vi "FlexMag - 23-03-2023.vi"() -> ()   [LabVIEW 2018] (continued)
        n5932 = Build Array(49152 ("element")) -> (w10400:i32[])
        n5933 = call "MB Serial Master Query Write Multiple Registers (poly).vi"("VISA resource name"=w10402, "Starting Address"=u16 320, "Registers"=w10400, "error in"=w10401, "Serial Parameters"=w10395) -> ("VISA resource name out"=w10406:refnum<visa-resource-name>, "error out"=w10407:errorcluster)  [unwired: 12 in, 1 out]
        n5934 = Build Array(49407 ("element")) -> (w10403:i32[])
        n5935 = call "MB Serial Master Query Write Multiple Registers (poly).vi"("VISA resource name"=w10406, "Starting Address"=u16 320, "Registers"=w10403, "error in"=w10407, "Serial Parameters"=w10395) -> ("VISA resource name out"=w10397:refnum<visa-resource-name>, "error out"=w10396:errorcluster)  [unwired: 12 in, 1 out]
      }
      frame 11 {
        w10417 = T15 {"Mode"=enum."RTU", "Slave Address"=1} ("Serial Parameters")
        n5936 = Type Cast(type=i16 0, x="TC2_AO1_bottom_limit_value") -> (*(type *) &x=w10409:i16)
        n5937 = Build Array(w10409) -> (w10410:i16[])
        n5938 = Increment(x=u16 166) -> (x+1=w10414:u16)
        n5939 = local write "TC2_AO1_bottom_limit_set"(FALSE ("TC2_AO1_bottom_limit_set")) -> ()
        n5940 = call "MB Serial Master Query Write Multiple Registers (poly).vi"("VISA resource name"=w10416, "Starting Address"=w10414, "Registers"=w10410, "error in"=w10415, "Serial Parameters"=w10417) -> ("VISA resource name out"=w10424:refnum<visa-resource-name>, "error out"=w10423:errorcluster)  [unwired: 12 in, 1 out]
        n5941 = Build Array(49152 ("element")) -> (w10422:i32[])
        n5942 = call "MB Serial Master Query Write Multiple Registers (poly).vi"("VISA resource name"=w10424, "Starting Address"=u16 320, "Registers"=w10422, "error in"=w10423, "Serial Parameters"=w10417) -> ("VISA resource name out"=w10428:refnum<visa-resource-name>, "error out"=w10429:errorcluster)  [unwired: 12 in, 1 out]
        n5943 = Build Array(49407 ("element")) -> (w10425:i32[])
        n5944 = call "MB Serial Master Query Write Multiple Registers (poly).vi"("VISA resource name"=w10428, "Starting Address"=u16 320, "Registers"=w10425, "error in"=w10429, "Serial Parameters"=w10417) -> ("VISA resource name out"=w10419:refnum<visa-resource-name>, "error out"=w10418:errorcluster)  [unwired: 12 in, 1 out]
      }
      frame 12 {
        w10439 = T15 {"Mode"=enum."RTU", "Slave Address"=1} ("Serial Parameters")
        n5945 = Type Cast(type=i16 0, x=sgl 0.0 ("TC1_AO1_bottom_limit_value 2")) -> (*(type *) &x=w10431:i16)
        n5946 = Build Array(w10431) -> (w10432:i16[])
        n5947 = Increment(x=u16 198) -> (x+1=w10436:u16)
        n5948 = local write "TC2_AO1_polarity(neg_to_pos)"(FALSE ("TC2_AO1_polarity(neg_to_pos)")) -> ()
        n5949 = call "MB Serial Master Query Write Multiple Registers (poly).vi"("VISA resource name"=w10438, "Starting Address"=w10436, "Registers"=w10432, "error in"=w10437, "Serial Parameters"=w10439) -> ("VISA resource name out"=w10446:refnum<visa-resource-name>, "error out"=w10445:errorcluster)  [unwired: 12 in, 1 out]
        n5950 = Build Array(49152 ("element")) -> (w10444:i32[])
        n5951 = call "MB Serial Master Query Write Multiple Registers (poly).vi"("VISA resource name"=w10446, "Starting Address"=u16 320, "Registers"=w10444, "error in"=w10445, "Serial Parameters"=w10439) -> ("VISA resource name out"=w10450:refnum<visa-resource-name>, "error out"=w10451:errorcluster)  [unwired: 12 in, 1 out]
        n5952 = Build Array(49407 ("element")) -> (w10447:i32[])
        n5953 = call "MB Serial Master Query Write Multiple Registers (poly).vi"("VISA resource name"=w10450, "Starting Address"=u16 320, "Registers"=w10447, "error in"=w10451, "Serial Parameters"=w10439) -> ("VISA resource name out"=w10441:refnum<visa-resource-name>, "error out"=w10440:errorcluster)  [unwired: 12 in, 1 out]
      }
      frame 13 {
        w10461 = T15 {"Mode"=enum."RTU", "Slave Address"=1} ("Serial Parameters")
        n5954 = Type Cast(type=i16 0, x=sgl 1.0 ("TC1_AO1_bottom_limit_value 2")) -> (*(type *) &x=w10453:i16)
        n5955 = Build Array(w10453) -> (w10454:i16[])
        n5956 = Increment(x=u16 198) -> (x+1=w10458:u16)
        n5957 = local write "TC2_AO1_polarity(pos_to_neg)"(FALSE ("TC2_AO1_polarity(pos_to_neg)")) -> ()
        n5958 = call "MB Serial Master Query Write Multiple Registers (poly).vi"("VISA resource name"=w10460, "Starting Address"=w10458, "Registers"=w10454, "error in"=w10459, "Serial Parameters"=w10461) -> ("VISA resource name out"=w10468:refnum<visa-resource-name>, "error out"=w10467:errorcluster)  [unwired: 12 in, 1 out]
        n5959 = Build Array(49152 ("element")) -> (w10466:i32[])
        n5960 = call "MB Serial Master Query Write Multiple Registers (poly).vi"("VISA resource name"=w10468, "Starting Address"=u16 320, "Registers"=w10466, "error in"=w10467, "Serial Parameters"=w10461) -> ("VISA resource name out"=w10472:refnum<visa-resource-name>, "error out"=w10473:errorcluster)  [unwired: 12 in, 1 out]
        n5961 = Build Array(49407 ("element")) -> (w10469:i32[])
        n5962 = call "MB Serial Master Query Write Multiple Registers (poly).vi"("VISA resource name"=w10472, "Starting Address"=u16 320, "Registers"=w10469, "error in"=w10473, "Serial Parameters"=w10461) -> ("VISA resource name out"=w10463:refnum<visa-resource-name>, "error out"=w10462:errorcluster)  [unwired: 12 in, 1 out]
      }
      frame 14 {
        w10483 = T15 {"Mode"=enum."RTU", "Slave Address"=1} ("Serial Parameters")
        n5963 = Type Cast(type=i16 0, x=sgl 2.0 ("TC1_AO1_bottom_limit_value 2")) -> (*(type *) &x=w10475:i16)
        n5964 = local write "TC2_display_tension_set"(FALSE ("TC2_display_tension")) -> ()
        n5965 = Build Array(w10475) -> (w10476:i16[])
        n5966 = Increment(x=u16 8) -> (x+1=w10480:u16)
        n5967 = call "MB Serial Master Query Write Multiple Registers (poly).vi"("VISA resource name"=w10482, "Starting Address"=w10480, "Registers"=w10476, "error in"=w10481, "Serial Parameters"=w10483) -> ("VISA resource name out"=w10490:refnum<visa-resource-name>, "error out"=w10489:errorcluster)  [unwired: 12 in, 1 out]
        n5968 = Build Array(49152 ("element")) -> (w10488:i32[])
        n5969 = call "MB Serial Master Query Write Multiple Registers (poly).vi"("VISA resource name"=w10490, "Starting Address"=u16 320, "Registers"=w10488, "error in"=w10489, "Serial Parameters"=w10483) -> ("VISA resource name out"=w10494:refnum<visa-resource-name>, "error out"=w10495:errorcluster)  [unwired: 12 in, 1 out]
        n5970 = Build Array(49407 ("element")) -> (w10491:i32[])
        n5971 = call "MB Serial Master Query Write Multiple Registers (poly).vi"("VISA resource name"=w10494, "Starting Address"=u16 320, "Registers"=w10491, "error in"=w10495, "Serial Parameters"=w10483) -> ("VISA resource name out"=w10485:refnum<visa-resource-name>, "error out"=w10484:errorcluster)  [unwired: 12 in, 1 out]
      }
      frame 15 {
        w10505 = T15 {"Mode"=enum."RTU", "Slave Address"=1} ("Serial Parameters")
        n5972 = Type Cast(type=i16 0, x=sgl 5.0 ("TC1_AO1_bottom_limit_value 2")) -> (*(type *) &x=w10497:i16)
        n5973 = Build Array(w10497) -> (w10498:i16[])
        n5974 = Increment(x=u16 8) -> (x+1=w10502:u16)
        n5975 = call "MB Serial Master Query Write Multiple Registers (poly).vi"("VISA resource name"=w10504, "Starting Address"=w10502, "Registers"=w10498, "error in"=w10503, "Serial Parameters"=w10505) -> ("VISA resource name out"=w10512:refnum<visa-resource-name>, "error out"=w10511:errorcluster)  [unwired: 12 in, 1 out]
        n5976 = local write "TC2_display_AO1_set"(FALSE ("TC2_display_tension")) -> ()
        n5977 = Build Array(49152 ("element")) -> (w10510:i32[])
        n5978 = call "MB Serial Master Query Write Multiple Registers (poly).vi"("VISA resource name"=w10512, "Starting Address"=u16 320, "Registers"=w10510, "error in"=w10511, "Serial Parameters"=w10505) -> ("VISA resource name out"=w10516:refnum<visa-resource-name>, "error out"=w10517:errorcluster)  [unwired: 12 in, 1 out]
        n5979 = Build Array(49407 ("element")) -> (w10513:i32[])
        n5980 = call "MB Serial Master Query Write Multiple Registers (poly).vi"("VISA resource name"=w10516, "Starting Address"=u16 320, "Registers"=w10513, "error in"=w10517, "Serial Parameters"=w10505) -> ("VISA resource name out"=w10507:refnum<visa-resource-name>, "error out"=w10506:errorcluster)  [unwired: 12 in, 1 out]
      }
      frame 16 {
        w10527 = T15 {"Mode"=enum."RTU", "Slave Address"=1} ("Serial Parameters")
        n5981 = Type Cast(type=i16 0, x=sgl 4.0 ("TC1_AO1_bottom_limit_value 2")) -> (*(type *) &x=w10519:i16)
        n5982 = local write "TC2_display_tension_actual"(FALSE ("TC2_display_tension")) -> ()
        n5983 = Build Array(w10519) -> (w10520:i16[])
        n5984 = Increment(x=u16 10) -> (x+1=w10524:u16)
        n5985 = call "MB Serial Master Query Write Multiple Registers (poly).vi"("VISA resource name"=w10526, "Starting Address"=w10524, "Registers"=w10520, "error in"=w10525, "Serial Parameters"=w10527) -> ("VISA resource name out"=w10534:refnum<visa-resource-name>, "error out"=w10533:errorcluster)  [unwired: 12 in, 1 out]
        n5986 = Build Array(49152 ("element")) -> (w10532:i32[])
        n5987 = call "MB Serial Master Query Write Multiple Registers (poly).vi"("VISA resource name"=w10534, "Starting Address"=u16 320, "Registers"=w10532, "error in"=w10533, "Serial Parameters"=w10527) -> ("VISA resource name out"=w10538:refnum<visa-resource-name>, "error out"=w10539:errorcluster)  [unwired: 12 in, 1 out]
        n5988 = Build Array(49407 ("element")) -> (w10535:i32[])
        n5989 = call "MB Serial Master Query Write Multiple Registers (poly).vi"("VISA resource name"=w10538, "Starting Address"=u16 320, "Registers"=w10535, "error in"=w10539, "Serial Parameters"=w10527) -> ("VISA resource name out"=w10529:refnum<visa-resource-name>, "error out"=w10528:errorcluster)  [unwired: 12 in, 1 out]
      }
      frame 17 {
        w10549 = T15 {"Mode"=enum."RTU", "Slave Address"=1} ("Serial Parameters")
        n5990 = Type Cast(type=i16 0, x=sgl 0.0 ("TC1_AO1_bottom_limit_value 2")) -> (*(type *) &x=w10541:i16)
        n5991 = Build Array(w10541) -> (w10542:i16[])
        n5992 = Increment(x=u16 10) -> (x+1=w10546:u16)
        n5993 = call "MB Serial Master Query Write Multiple Registers (poly).vi"("VISA resource name"=w10548, "Starting Address"=w10546, "Registers"=w10542, "error in"=w10547, "Serial Parameters"=w10549) -> ("VISA resource name out"=w10556:refnum<visa-resource-name>, "error out"=w10555:errorcluster)  [unwired: 12 in, 1 out]
        n5994 = local write "TC2_display_AO1_actual"(FALSE ("TC2_display_tension")) -> ()
        n5995 = Build Array(49152 ("element")) -> (w10554:i32[])
        n5996 = call "MB Serial Master Query Write Multiple Registers (poly).vi"("VISA resource name"=w10556, "Starting Address"=u16 320, "Registers"=w10554, "error in"=w10555, "Serial Parameters"=w10549) -> ("VISA resource name out"=w10560:refnum<visa-resource-name>, "error out"=w10561:errorcluster)  [unwired: 12 in, 1 out]
        n5997 = Build Array(49407 ("element")) -> (w10557:i32[])
        n5998 = call "MB Serial Master Query Write Multiple Registers (poly).vi"("VISA resource name"=w10560, "Starting Address"=u16 320, "Registers"=w10557, "error in"=w10561, "Serial Parameters"=w10549) -> ("VISA resource name out"=w10551:refnum<visa-resource-name>, "error out"=w10550:errorcluster)  [unwired: 12 in, 1 out]
      }
      frame 18 {
        n5999 = Build Array(i16 21767) -> (w10568:i16[])
        n6000 = call "MB Serial Master Query Write Multiple Registers (poly).vi"("VISA resource name"=w10570, "Starting Address"=u16 322 ("x"), "Registers"=w10568, "error in"=w10569, "Serial Parameters"=T15 {"Mode"=enum."RTU", "Slave Address"=1}) -> ("VISA resource name out"=w10563:refnum<visa-resource-name>, "error out"=w10564:errorcluster)  [unwired: 12 in, 1 out]
        n6001 = local write "TC2_tare_function"(FALSE ("TC2_tare_function")) -> ()
        n6002 = Build Array(49407 ("element")) -> (w10573:i32[])
        n6003 = call "MB Serial Master Query Write Multiple Registers (poly).vi"("VISA resource name"=w10563, "Starting Address"=u16 320, "Registers"=w10573, "error in"=w10564) -> ("VISA resource name out"=w10572:refnum<visa-resource-name>, "error out"=w10571:errorcluster)  [unwired: 13 in, 1 out]
      }
      frame 19 {
        w10594 = T15 {"Mode"=enum."RTU", "Slave Address"=1} ("Serial Parameters")
        n6004 = Build Array("TC2_regulation_type_value") -> (w10583:sgl[])
        n6005 = call "MB Serial Master Query Write Multiple Registers (poly).vi"("VISA resource name"=w10580, "Starting Address"=u16 107, "Registers"=w10583, "error in"=w10579, "Serial Parameters"=w10594) -> ("VISA resource name out"=w10592:refnum<visa-resource-name>, "error out"=w10593:errorcluster)  [unwired: 12 in, 1 out]
        n6006 = Build Array(49152 ("element")) -> (w10587:i32[])
        n6007 = local write "TC2_regulation_type_selection"(FALSE ("TC2_regulation_type_selection")) -> ()
        n6008 = call "MB Serial Master Query Write Multiple Registers (poly).vi"("VISA resource name"=w10592, "Starting Address"=u16 320, "Registers"=w10587, "error in"=w10593, "Serial Parameters"=w10594) -> ("VISA resource name out"=w10585:refnum<visa-resource-name>, "error out"=w10584:errorcluster)  [unwired: 12 in, 1 out]
        n6009 = Build Array(49407 ("element")) -> (w10586:i32[])
        n6010 = call "MB Serial Master Query Write Multiple Registers (poly).vi"("VISA resource name"=w10585, "Starting Address"=u16 320, "Registers"=w10586, "error in"=w10584, "Serial Parameters"=w10594) -> ("VISA resource name out"=w10581:refnum<visa-resource-name>, "error out"=w10578:errorcluster)  [unwired: 12 in, 1 out]
      }
      frame 20 {
        w10613 = T15 {"Mode"=enum."RTU", "Slave Address"=1} ("Serial Parameters")
        n6011 = Build Array("TC2_setpoint_type_value") -> (w10602:sgl[])
        n6012 = call "MB Serial Master Query Write Multiple Registers (poly).vi"("VISA resource name"=w10599, "Starting Address"=u16 141, "Registers"=w10602, "error in"=w10598, "Serial Parameters"=w10613) -> ("VISA resource name out"=w10611:refnum<visa-resource-name>, "error out"=w10612:errorcluster)  [unwired: 12 in, 1 out]
        n6013 = Build Array(49152 ("element")) -> (w10606:i32[])
        n6014 = call "MB Serial Master Query Write Multiple Registers (poly).vi"("VISA resource name"=w10611, "Starting Address"=u16 320, "Registers"=w10606, "error in"=w10612, "Serial Parameters"=w10613) -> ("VISA resource name out"=w10604:refnum<visa-resource-name>, "error out"=w10603:errorcluster)  [unwired: 12 in, 1 out]
        n6015 = local write "TC2_setpoint_type"(FALSE ("TC2_regulation_type_selection")) -> ()
        n6016 = Build Array(49407 ("element")) -> (w10605:i32[])
        n6017 = call "MB Serial Master Query Write Multiple Registers (poly).vi"("VISA resource name"=w10604, "Starting Address"=u16 320, "Registers"=w10605, "error in"=w10603, "Serial Parameters"=w10613) -> ("VISA resource name out"=w10600:refnum<visa-resource-name>, "error out"=w10597:errorcluster)  [unwired: 12 in, 1 out]
      }
      frame 21 {
        w10632 = T15 {"Mode"=enum."RTU", "Slave Address"=1} ("Serial Parameters")
        n6018 = Build Array("tc2 data set to reg") -> (w10621:sgl[])
        n6019 = call "MB Serial Master Query Write Multiple Registers (poly).vi"("VISA resource name"=w10619, "Starting Address"="tc2 Starting Address", "Registers"=w10621, "error in"=w10618, "Serial Parameters"=w10632) -> ("VISA resource name out"=w10630:refnum<visa-resource-name>, "error out"=w10631:errorcluster)  [unwired: 12 in, 1 out]
        n6020 = Build Array(49152 ("element")) -> (w10625:i32[])
        n6021 = call "MB Serial Master Query Write Multiple Registers (poly).vi"("VISA resource name"=w10630, "Starting Address"=u16 320, "Registers"=w10625, "error in"=w10631, "Serial Parameters"=w10632) -> ("VISA resource name out"=w10623:refnum<visa-resource-name>, "error out"=w10622:errorcluster)  [unwired: 12 in, 1 out]
        n6022 = local write "TC2_reg_set"(FALSE ("TC2_regulation_type_selection")) -> ()
        n6023 = Build Array(49407 ("element")) -> (w10624:i32[])
        n6024 = call "MB Serial Master Query Write Multiple Registers (poly).vi"("VISA resource name"=w10623, "Starting Address"=u16 320, "Registers"=w10624, "error in"=w10622, "Serial Parameters"=w10632) -> ("VISA resource name out"=w10620:refnum<visa-resource-name>, "error out"=w10617:errorcluster)  [unwired: 12 in, 1 out]
      }
    }
  }
  n6025 = while {
    tunnel: w45 -> [w11141]
    tunnel: w44 -> [w11140]
    tunnel: [w11139] -> w43
    tunnel: [w11138] -> w42
    stop <- FALSE stop-if-true
    n6026 = Wait Until Next ms Multiple(millisecond multiple=u32 300) -> ()  [unwired: 1 out]
    n6027 = case shown="False" "Counter data set" {
      tunnel: w11141 -> [w11149 w11158]
      tunnel: [w11148 w11157] -> w11139
      tunnel: [w11147 w11156] -> w11138
      tunnel: w11140 -> [w11143 _]
      frame False {
        n6028 = call-poly "MB Serial Master Query (poly).vi"("VISA resource name"=w11149, "Starting Address"=u16 1000, "Quantity"=u16 13, "error in"=w11143, "Serial Parameters"=T15 {"Mode"=enum."RTU", "Slave Address"=1}) -> ("VISA resource name out"=w11148:refnum<visa-resource-name>, "Input Registers"=w11146:u16[], "error out"=w11147:errorcluster)  [unwired: 1 in, 11 out]
        n6029 = Index Array(array=w11146, index=3) -> (element=→"Counter Read Data":u16)
      }
      frame True {
        n6030 = local write "Counter data set"(FALSE ("Counter_reset")) -> ()
        n6031 = call-poly "MB Serial Master Query (poly).vi"("VISA resource name"=w11158, "Address"="Counter Data set", "Coil"=TRUE, "Serial Parameters"=T15 {"Mode"=enum."RTU", "Slave Address"=1}) -> ("VISA resource name out"=w11157:refnum<visa-resource-name>, "error out"=w11156:errorcluster)  [unwired: 2 in, 12 out]
      }
    }
  }
  n6032 = while {
    tunnel: w27 -> [w11175]
    tunnel: w26 -> [w11174]
    tunnel: [w11172] -> w28
    tunnel: [w11171] -> w29
    stop <- FALSE stop-if-true
    n6033 = Compound Arithmetic op=OR("MWPS1 open", "MWPS1 auto open") -> (w11161:bool)
    n6034 = Compound Arithmetic op=OR("MWPS1 close", "MWPS1 auto close") -> (w11160:bool)
    n6035 = Wait Until Next ms Multiple(millisecond multiple=u32 300) -> ()  [unwired: 1 out]
    n6036 = Build Array(FALSE, w11161, w11160) -> (w11168:bool[])
    n6037 = Boolean Array To Number(Boolean array=w11168) -> (number=w11167:u32)
    n6038 = Mantissa & Exponent(0:w11167) -> (2:w11166:dbl)  [unwired: 1 out]
    n6039 = case shown="1" w11166 {
      tunnel: w11175 -> [w11190 w11222 w11242]
      tunnel: w11174 -> [w11189 w11221 w11241]
      tunnel: [w11188 w11212 w11232] -> w11172
      tunnel: [w11187 w11211 w11231] -> w11171
      frame 0, Default {
        n6040 = VISA Write(VISA resource name=w11190, write buffer="\u0000%\u0000%", error in (no error)=w11189) -> (VISA resource name out=w11186:refnum<visa-resource-name>, error out=w11185:errorcluster)  [unwired: 1 out]
        n6041 = property class="Instr"(reference=w11186, error in=w11185) -> (reference out=w11184:refnum<visa-resource-name>, error out=w11183:errorcluster, "Serial Settings:Number of Bytes at Serial Port"=w11182:u32)
        n6042 = stacked-sequence {
          tunnel: [w11194] -> w11181
          tunnel: w11184 -> [w11194]
          tunnel: [w11193] -> w11180
          tunnel: w11183 -> [w11193]
          tunnel: [w11192] -> w11179
          tunnel: w11182 -> [w11192]
          tunnel: "microwave1 wait ms" -> [w11191]
          frame #0 {
            n6043 = Wait (ms)(milliseconds to wait=w11191) -> ()  [unwired: 1 out]
          }
        }
        n6044 = VISA Read(VISA resource name=w11181, byte count=w11179, error in (no error)=w11180) -> (VISA resource name out=w11188:refnum<visa-resource-name>, read buffer=→"microwave1 read":string, error out=w11187:errorcluster)  [unwired: 1 out]
      }
      frame 1 {
        n6045 = stacked-sequence {
          frame #0 {
            n6046 = Wait (ms)(milliseconds to wait=u32 200) -> ()  [unwired: 1 out]
          }
          frame #1 {
            n6047 = local write "MWPS1 auto open"(FALSE ("Mwps_auto_open")) -> ()
          }
        }
        n6048 = Divide(x="MWPS1 set", y=10.0) -> (x/y=w11205:dbl)
        n6049 = Add(x=w11205, y=165.0 ("Mwps_set 2")) -> (x+y=w11199:dbl)
        n6050 = Greater?(x=w11199, y=256.0) -> (0:w11203:bool)
        n6051 = Subtract(x=w11199, y=256.0) -> (x-y=w11200:dbl)
        n6052 = Select(t=w11200, s=w11203, f=w11199) -> (s? t:f=w11197:dbl)
        n6053 = Build Array(w11205) -> (w11209:dbl[])
        n6054 = Build Array(w11197) -> (w11198:dbl[])
        n6055 = Byte Array To String(unsigned byte array=w11209) -> (string=w11208:string)
        n6056 = Byte Array To String(unsigned byte array=w11198) -> (string=w11196:string)
        n6057 = Concatenate Strings("€%" ("write buffer"), w11208, w11196) -> (w11195:string)
        n6058 = VISA Write(VISA resource name=w11222, write buffer=w11195, error in (no error)=w11221) -> (VISA resource name out=w11220:refnum<visa-resource-name>, error out=w11219:errorcluster)  [unwired: 1 out]
        n6059 = property class="Instr"(reference=w11220, error in=w11219) -> (reference out=w11218:refnum<visa-resource-name>, error out=w11217:errorcluster, "Serial Settings:Number of Bytes at Serial Port"=w11216:u32)
        n6060 = stacked-sequence {
          tunnel: [w11228] -> w11215
          tunnel: w11218 -> [w11228]
          tunnel: [w11227] -> w11214
          tunnel: w11217 -> [w11227]
          tunnel: [w11226] -> w11213
          tunnel: w11216 -> [w11226]
          frame #0 {
            n6061 = Wait (ms)(milliseconds to wait=u32 300) -> ()  [unwired: 1 out]
          }
        }
        n6062 = VISA Read(VISA resource name=w11215, byte count=w11213, error in (no error)=w11214) -> (VISA resource name out=w11212:refnum<visa-resource-name>, error out=w11211:errorcluster)  [unwired: 2 out]
      }
      frame 2 {
        n6063 = stacked-sequence {
          frame #0 {
            n6064 = Wait (ms)(milliseconds to wait=u32 200) -> ()  [unwired: 1 out]
          }
          frame #1 {
            n6065 = local write "MWPS1 auto close"(FALSE ("Mwps_auto_open")) -> ()
          }
        }
        n6066 = local write "MWPS1 set"(0.0 ("Mwps_set")) -> ()
        n6067 = VISA Write(VISA resource name=w11242, write buffer="€%\u0000¥", error in (no error)=w11241) -> (VISA resource name out=w11240:refnum<visa-resource-name>, error out=w11239:errorcluster)  [unwired: 1 out]
        n6068 = property class="Instr"(reference=w11240, error in=w11239) -> (reference out=w11238:refnum<visa-resource-name>, error out=w11237:errorcluster, "Serial Settings:Number of Bytes at Serial Port"=w11236:u32)
        n6069 = stacked-sequence {
          tunnel: [w11248] -> w11235
          tunnel: w11238 -> [w11248]
          tunnel: [w11247] -> w11234
          tunnel: w11237 -> [w11247]
          tunnel: [w11246] -> w11233
          tunnel: w11236 -> [w11246]
          frame #0 {
            n6070 = Wait (ms)(milliseconds to wait=u32 300) -> ()  [unwired: 1 out]
          }
        }
        n6071 = VISA Read(VISA resource name=w11235, byte count=w11233, error in (no error)=w11234) -> (VISA resource name out=w11232:refnum<visa-resource-name>, error out=w11231:errorcluster)  [unwired: 2 out]
      }
    }
  }
  n6072 = while {
    tunnel: w24 -> [w11264]
    tunnel: w25 -> [w11263]
    tunnel: [w11261] -> w22
    tunnel: [w11260] -> w23
    stop <- FALSE stop-if-true
    n6073 = Wait Until Next ms Multiple(millisecond multiple=u32 300) -> ()  [unwired: 1 out]
    n6074 = Compound Arithmetic op=OR("MWPS2 open", "MWPS2 auto open") -> (w11249:bool)
    n6075 = Compound Arithmetic op=OR("MWPS2 close", "MWPS2 auto close") -> (w11250:bool)
    n6076 = Build Array(FALSE, w11249, w11250) -> (w11257:bool[])
    n6077 = Boolean Array To Number(Boolean array=w11257) -> (number=w11256:u32)
    n6078 = Mantissa & Exponent(0:w11256) -> (2:w11255:dbl)  [unwired: 1 out]
    n6079 = case shown="0, Default" w11255 {
      tunnel: w11264 -> [w11279 w11311 w11331]
      tunnel: w11263 -> [w11278 w11310 w11330]
      tunnel: [w11277 w11301 w11321] -> w11261
      tunnel: [w11276 w11300 w11320] -> w11260
      frame 0, Default {
        n6080 = VISA Write(VISA resource name=w11279, write buffer="\u0000%\u0000%", error in (no error)=w11278) -> (VISA resource name out=w11275:refnum<visa-resource-name>, error out=w11274:errorcluster)  [unwired: 1 out]
        n6081 = property class="Instr"(reference=w11275, error in=w11274) -> (reference out=w11273:refnum<visa-resource-name>, error out=w11272:errorcluster, "Serial Settings:Number of Bytes at Serial Port"=w11271:u32)
        n6082 = stacked-sequence {
          tunnel: [w11283] -> w11270
          tunnel: w11273 -> [w11283]
          tunnel: [w11282] -> w11269
          tunnel: w11272 -> [w11282]
          tunnel: [w11281] -> w11268
          tunnel: w11271 -> [w11281]
          tunnel: "microwave2 wait ms" -> [w11280]
          frame #0 {
            n6083 = Wait (ms)(milliseconds to wait=w11280) -> ()  [unwired: 1 out]
          }
        }
        n6084 = VISA Read(VISA resource name=w11270, byte count=w11268, error in (no error)=w11269) -> (VISA resource name out=w11277:refnum<visa-resource-name>, read buffer=→"microwave2 read":string, error out=w11276:errorcluster)  [unwired: 1 out]
      }
      frame 1 {
        n6085 = stacked-sequence {
          frame #0 {
            n6086 = Wait (ms)(milliseconds to wait=u32 200) -> ()  [unwired: 1 out]
          }
          frame #1 {
            n6087 = local write "MWPS2 auto open"(FALSE ("Mwps_auto_open")) -> ()
          }
        }
        n6088 = Divide(x="MWPS2 set", y=10.0) -> (x/y=w11294:dbl)
        n6089 = Add(x=w11294, y=165.0 ("Mwps_set 2")) -> (x+y=w11288:dbl)
        n6090 = Greater?(x=w11288, y=256.0) -> (0:w11292:bool)
        n6091 = Subtract(x=w11288, y=256.0) -> (x-y=w11289:dbl)
        n6092 = Select(t=w11289, s=w11292, f=w11288) -> (s? t:f=w11286:dbl)
        n6093 = Build Array(w11294) -> (w11298:dbl[])
        n6094 = Build Array(w11286) -> (w11287:dbl[])
        n6095 = Byte Array To String(unsigned byte array=w11298) -> (string=w11297:string)
        n6096 = Byte Array To String(unsigned byte array=w11287) -> (string=w11285:string)
        n6097 = Concatenate Strings("€%" ("write buffer"), w11297, w11285) -> (w11284:string)
        n6098 = VISA Write(VISA resource name=w11311, write buffer=w11284, error in (no error)=w11310) -> (VISA resource name out=w11309:refnum<visa-resource-name>, error out=w11308:errorcluster)  [unwired: 1 out]
        n6099 = property class="Instr"(reference=w11309, error in=w11308) -> (reference out=w11307:refnum<visa-resource-name>, error out=w11306:errorcluster, "Serial Settings:Number of Bytes at Serial Port"=w11305:u32)
        n6100 = stacked-sequence {
          tunnel: [w11317] -> w11304
          tunnel: w11307 -> [w11317]
          tunnel: [w11316] -> w11303
          tunnel: w11306 -> [w11316]
          tunnel: [w11315] -> w11302
          tunnel: w11305 -> [w11315]
          frame #0 {
            n6101 = Wait (ms)(milliseconds to wait=u32 300) -> ()  [unwired: 1 out]
          }
        }
        n6102 = VISA Read(VISA resource name=w11304, byte count=w11302, error in (no error)=w11303) -> (VISA resource name out=w11301:refnum<visa-resource-name>, error out=w11300:errorcluster)  [unwired: 2 out]
      }
      frame 2 {
        n6103 = stacked-sequence {
          frame #0 {
            n6104 = Wait (ms)(milliseconds to wait=u32 200) -> ()  [unwired: 1 out]
          }
          frame #1 {
            n6105 = local write "MWPS2 auto close"(FALSE ("Mwps_auto_open")) -> ()
          }
        }
        n6106 = local write "MWPS2 set"(0.0 ("Mwps_set")) -> ()
        n6107 = VISA Write(VISA resource name=w11331, write buffer="€%\u0000¥", error in (no error)=w11330) -> (VISA resource name out=w11329:refnum<visa-resource-name>, error out=w11328:errorcluster)  [unwired: 1 out]
        n6108 = property class="Instr"(reference=w11329, error in=w11328) -> (reference out=w11327:refnum<visa-resource-name>, error out=w11326:errorcluster, "Serial Settings:Number of Bytes at Serial Port"=w11325:u32)
        n6109 = stacked-sequence {
          tunnel: [w11337] -> w11324
          tunnel: w11327 -> [w11337]
          tunnel: [w11336] -> w11323
          tunnel: w11326 -> [w11336]
          tunnel: [w11335] -> w11322
          tunnel: w11325 -> [w11335]
          frame #0 {
            n6110 = Wait (ms)(milliseconds to wait=u32 300) -> ()  [unwired: 1 out]
          }
        }
        n6111 = VISA Read(VISA resource name=w11324, byte count=w11322, error in (no error)=w11323) -> (VISA resource name out=w11321:refnum<visa-resource-name>, error out=w11320:errorcluster)  [unwired: 2 out]
      }
    }
  }
  n6112 = while {
    tunnel: w58 -> [w11763]
    tunnel: w59 -> [w11762]
    shift-right: [w11588] -> _
    shift-left: _ -> [w11587]
    tunnel: [w11511] -> w60
    tunnel: [w11510] -> w61
    stop <- FALSE stop-if-true
    w11401 = "\b—"
    w11363 = "\b¢"
    # "guc kaynagı ACK gelınceye kadar bekler."
    # "ACK karsılıgı 06(hex) dır."
    n6113 = Tick Count (ms)() -> (millisecond timer value=w11588:u32)
    n6114 = Or(x="set rf", y="RF_auto_set") -> (x .or. y?=w11347:bool)
    n6115 = Or(x="RF on", y="RF_auto_on") -> (x .or. y?=w11358:bool)
    n6116 = Or(x="oto tuner", y="RF_auto_tuner") -> (x .or. y?=w11339:bool)
    n6117 = Or(x="RF off", y="RF_auto_off") -> (x .or. y?=w11356:bool)
    n6118 = Or(x="RF host", y="RF_auto_host") -> (x .or. y?=w11353:bool)
    n6119 = Subtract(x=w11588, y=w11587) -> (x-y=→"x-y":u32)
    n6120 = Or(x="Ramp Up time", y="Ramp Up time_auto") -> (x .or. y?=w11351:bool)
    n6121 = Boolean To (0,1)(Boolean=w11353) -> (0, 1=w11737:i16)
    n6122 = Boolean To (0,1)(Boolean=w11356) -> (0, 1=w11738:i16)
    n6123 = Boolean To (0,1)(Boolean=w11358) -> (0, 1=w11744:i16)
    n6124 = Boolean To (0,1)(Boolean=w11347) -> (0, 1=w11743:i16)
    n6125 = Boolean To (0,1)(Boolean=w11339) -> (0, 1=w11742:i16)
    n6126 = Boolean To (0,1)(Boolean="initialize") -> (0, 1=w11740:i16)
    n6127 = Boolean To (0,1)(Boolean="Load") -> (0, 1=w11465:i16)
    n6128 = Boolean To (0,1)(Boolean="Forward") -> (0, 1=w11462:i16)
    n6129 = Boolean To (0,1)(Boolean="External") -> (0, 1=w11468:i16)
    n6130 = Boolean To (0,1)(Boolean="Pulsing_off") -> (0, 1=w11475:i16)
    n6131 = Boolean To (0,1)(Boolean="internal") -> (0, 1=w11476:i16)
    n6132 = Boolean To (0,1)(Boolean="external") -> (0, 1=w11478:i16)
    n6133 = Boolean To (0,1)(Boolean="set duty") -> (0, 1=w11491:i16)
    n6134 = Boolean To (0,1)(Boolean=w11351) -> (0, 1=w11450:i16)
    n6135 = Boolean To (0,1)(Boolean="manuel tuner") -> (0, 1=w11741:i16)
    n6136 = Boolean To (0,1)(Boolean="set cap pos") -> (0, 1=w11739:i16)
    n6137 = Boolean To (0,1)(Boolean="set seri cap pos 2") -> (0, 1=w11736:i16)
    n6138 = Boolean To (0,1)(Boolean="set frequency") -> (0, 1=w11487:i16)
    n6139 = Multiply(x=w11737, y=i16 1) -> (x*y=w11460:i16)
    n6140 = Multiply(x=w11738, y=i16 3) -> (x*y=w11757:i16)
    n6141 = Multiply(x=w11744, y=i16 4) -> (x*y=w11758:i16)
    n6142 = Multiply(x=w11743, y=i16 5) -> (x*y=w11755:i16)
    n6143 = Multiply(x=w11742, y=i16 6) -> (x*y=w11753:i16)
    n6144 = Multiply(x=w11740, y=i16 8) -> (x*y=w11749:i16)
    n6145 = Or(x="Ramp down time", y="Ramp Down time_auto") -> (x .or. y?=w11346:bool)
    n6146 = Boolean To (0,1)(Boolean=w11346) -> (0, 1=w11448:i16)
    n6147 = Multiply(x=w11741, y=i16 7) -> (x*y=w11751:i16)
    n6148 = Multiply(x=w11739, y=i16 9) -> (x*y=w11747:i16)
    n6149 = Multiply(x=w11465, y=i16 2) -> (x*y=w11485:i16)
    n6150 = Multiply(x=w11736, y=i16 10) -> (x*y=w11745:i16)
    n6151 = Multiply(x=w11462, y=i16 11) -> (x*y=w11484:i16)
    n6152 = Multiply(x=w11468, y=i16 12) -> (x*y=w11483:i16)
    n6153 = Multiply(x=w11475, y=i16 13) -> (x*y=w11480:i16)
    n6154 = Multiply(x=w11476, y=i16 14) -> (x*y=w11481:i16)
    n6155 = Multiply(x=w11478, y=i16 15) -> (x*y=w11482:i16)
    n6156 = Multiply(x=w11487, y=i16 16) -> (x*y=w11489:i16)
    n6157 = Multiply(x=w11491, y=i16 17) -> (x*y=w11493:i16)
    n6158 = Multiply(x=w11450, y=i16 18) -> (x*y=w11447:i16)
    n6159 = Multiply(x=w11448, y=i16 19) -> (x*y=w11446:i16)
    n6160 = String To Byte Array(string=w11363) -> (unsigned byte array=w11445:u8[])
    n6161 = for {
      tunnel: w11445 -> [w11799] mode=indexing
      shift-right: [w11797] -> w11443
      shift-left: 0 -> [w11798]
      n6162 = Exclusive Or(1:w11798, 2:w11799) -> (0:w11797:i32)
    }
    n6163 = Wait Until Next ms Multiple(millisecond multiple=u32 300) -> ()  [unwired: 1 out]
    n6164 = Compound Arithmetic op=ADD(w11485, w11484, w11483, w11480, w11481, w11482, w11489, w11493) -> (w11461:i16)
    n6165 = Build Array(w11443) -> (w11442:i32[])
    n6166 = Compound Arithmetic op=ADD(w11460, w11757, w11758, w11755, w11753, w11751, w11749, w11747, w11745, w11461, w11447, w11446) -> (w11733:i16)
    n6167 = Byte Array To String(unsigned byte array=w11442) -> (string=w11441:string)
    n6168 = case shown="5" w11733 {
      tunnel: [w11910 w11914 w11919 w11933 w11939 w11946 w11969 w11986 w12002 w12022 w12047 w12063 w12077 w12091 w12105 w12119 w12133 w12161 w12180 w12206] -> w11735
      tunnel: [w11909 w11913 w11918 w11934 w11940 w11947 w11968 w11985 w12003 w12021 w12046 w12062 w12076 w12090 w12104 w12118 w12132 w12160 w12179 w12205] -> w11734
      tunnel: w11763 -> [w11910 w11912 w11921 w11936 w11942 w11949 w11971 w11988 w12001 w12024 w12049 w12065 w12079 w12093 w12107 w12121 w12135 w12163 w12182 w12208]
      tunnel: w11762 -> [w11909 w11911 w11920 w11935 w11941 w11948 w11970 w11987 w12000 w12023 w12048 w12064 w12078 w12092 w12106 w12120 w12134 w12162 w12181 w12207]
      frame 0, Default {
      }
      frame 1 {
        # "Host kontrol"
        n6169 = flat-sequence {
          frame #0 {
            n6170 = Wait (ms)(milliseconds to wait=u32 200) -> ()  [unwired: 1 out]
          }
          frame #1 {
            n6171 = local write "RF_auto_host"(FALSE ("RF_host_auto")) -> ()
          }
        }
        n6172 = VISA Write(VISA resource name=w11912, write buffer="\t\u000e\u0002\u0005", error in (no error)=w11911) -> (VISA resource name out=w11914:refnum<visa-resource-name>, error out=w11913:errorcluster)  [unwired: 1 out]
      }
      frame 2 {
        w11928 = "\t\u0003\u0007"
        n6173 = String To Byte Array(string=w11928) -> (unsigned byte array=w11922:u8[])
        n6174 = for {
          tunnel: w11922 -> [w11931] mode=indexing
          shift-right: [w11929] -> w11924
          shift-left: 0 -> [w11930]
          n6175 = Exclusive Or(1:w11930, 2:w11931) -> (0:w11929:i32)
        }
        n6176 = Build Array(w11924) -> (w11926:i32[])
        n6177 = Byte Array To String(unsigned byte array=w11926) -> (string=w11925:string)
        n6178 = Concatenate Strings(w11928, w11925) -> (w11927:string)
        n6179 = VISA Write(VISA resource name=w11921, write buffer=w11927, error in (no error)=w11920) -> (VISA resource name out=w11919:refnum<visa-resource-name>, error out=w11918:errorcluster)  [unwired: 1 out]
      }
      frame 3 {
        # "RF OFF"
        n6180 = local write "RF_auto_off"(FALSE ("RF_auto_off")) -> ()
        n6181 = VISA Write(VISA resource name=w11936, write buffer="\b\u0001\t", error in (no error)=w11935) -> (VISA resource name out=w11933:refnum<visa-resource-name>, error out=w11934:errorcluster)  [unwired: 1 out]
      }
      frame 4 {
        # "RF ON"
        n6182 = local write "RF_auto_on"(FALSE ("RF_auto_on")) -> ()
        n6183 = VISA Write(VISA resource name=w11942, write buffer="\b\u0002\n", error in (no error)=w11941) -> (VISA resource name out=w11939:refnum<visa-resource-name>, error out=w11940:errorcluster)  [unwired: 1 out]
      }
      frame 5 {
        n6184 = Quotient & Remainder(x="RF_forward_power_1", y=256.0) -> (x-y*floor(x/y)=w11956:dbl, floor(x/y)=w11952:dbl)
        n6185 = Build Array(w11956) -> (w11955:dbl[])
        n6186 = Build Array(w11952) -> (w11953:dbl[])
        n6187 = Byte Array To String(unsigned byte array=w11955) -> (string=w11954:string)
        n6188 = Byte Array To String(unsigned byte array=w11953) -> (string=w11951:string)
        n6189 = Concatenate Strings("\n\b", w11954, w11951) -> (w11958:string)
        n6190 = String To Byte Array(string=w11958) -> (unsigned byte array=w11964:u8[])
        n6191 = for {
          tunnel: w11964 -> [w11967] mode=indexing
          shift-right: [w11965] -> w11962
          shift-left: 0 -> [w11966]
          n6192 = Exclusive Or(1:w11966, 2:w11967) -> (0:w11965:i32)
        }
        n6193 = local write "RF_auto_set"(FALSE ("RF set auto")) -> ()
        n6194 = Build Array(w11962) -> (w11961:i32[])
        n6195 = Byte Array To String(unsigned byte array=w11961) -> (string=w11959:string)
        n6196 = Concatenate Strings(w11958, w11959) -> (w11950:string)
        n6197 = VISA Write(VISA resource name=w11949, write buffer=w11950, error in (no error)=w11948) -> (VISA resource name out=w11946:refnum<visa-resource-name>, error out=w11947:errorcluster)  [unwired: 1 out]
      }
      frame 6 {
        n6198 = Concatenate Strings("\t\r\u0001") -> (w11973:string)
        n6199 = String To Byte Array(string=w11973) -> (unsigned byte array=w11979:u8[])
        n6200 = flat-sequence {
          frame #0 {
            n6201 = Wait (ms)(milliseconds to wait=u32 200) -> ()  [unwired: 1 out]
          }
          frame #1 {
            n6202 = local write "RF_auto_tuner"(FALSE ("RF_auto_tuner")) -> ()
          }
        }
        n6203 = for {
          tunnel: w11979 -> [w11984] mode=indexing
          shift-right: [w11982] -> w11977
          shift-left: 0 -> [w11983]
          n6204 = Exclusive Or(1:w11983, 2:w11984) -> (0:w11982:i32)
        }
        n6205 = Build Array(w11977) -> (w11976:i32[])
        n6206 = Byte Array To String(unsigned byte array=w11976) -> (string=w11974:string)
        n6207 = Concatenate Strings(w11973, w11974) -> (w11972:string)
        n6208 = VISA Write(VISA resource name=w11971, write buffer=w11972, error in (no error)=w11970) -> (VISA resource name out=w11969:refnum<visa-resource-name>, error out=w11968:errorcluster)  [unwired: 1 out]
      }
      frame 7 {
        n6209 = Concatenate Strings("\t\r\u0000") -> (w11990:string)
        n6210 = String To Byte Array(string=w11990) -> (unsigned byte array=w11996:u8[])
        n6211 = for {
          tunnel: w11996 -> [w11999] mode=indexing
          shift-right: [w11997] -> w11994
          shift-left: 0 -> [w11998]
          n6212 = Exclusive Or(1:w11998, 2:w11999) -> (0:w11997:i32)
        }
        n6213 = Build Array(w11994) -> (w11993:i32[])
        n6214 = Byte Array To String(unsigned byte array=w11993) -> (string=w11991:string)
        n6215 = Concatenate Strings(w11990, w11991) -> (w11989:string)
        n6216 = VISA Write(VISA resource name=w11988, write buffer=w11989, error in (no error)=w11987) -> (VISA resource name out=w11986:refnum<visa-resource-name>, error out=w11985:errorcluster)  [unwired: 1 out]
      }
      frame 8 {
        w12007 = "\bo"
        n6217 = String To Byte Array(string=w12007) -> (unsigned byte array=w12010:u8[])
        n6218 = for {
          tunnel: w12010 -> [w12013] mode=indexing
          shift-right: [w12011] -> w12008
          shift-left: 0 -> [w12012]
          n6219 = Exclusive Or(1:w12012, 2:w12013) -> (0:w12011:i32)
        }
        n6220 = Build Array(w12008) -> (w12005:i32[])
        n6221 = Byte Array To String(unsigned byte array=w12005) -> (string=w12006:string)
        n6222 = Concatenate Strings(w12007, w12006) -> (w12004:string)
        n6223 = VISA Write(VISA resource name=w12001, write buffer=w12004, error in (no error)=w12000) -> (VISA resource name out=w12002:refnum<visa-resource-name>, error out=w12003:errorcluster)  [unwired: 1 out]
      }
      frame 9 {
        n6224 = Multiply(x="Set CL Position:", y=10.0) -> (x*y=w12016:dbl)
        n6225 = To Unsigned Long Integer(number=w12016) -> (unsigned 32bit integer=w12015:u32)
        n6226 = Quotient & Remainder(x=w12015, y=u32 256) -> (x-y*floor(x/y)=w12020:u32, floor(x/y)=w12019:u32)
        n6227 = Build Array(w12020, w12019) -> (w12027:u32[])
        n6228 = Byte Array To String(unsigned byte array=w12027) -> (string=w12026:string)
        n6229 = Concatenate Strings("\np", w12026) -> (w12028:string)
        n6230 = String To Byte Array(string=w12028) -> (unsigned byte array=w12034:u8[])
        n6231 = for {
          tunnel: w12034 -> [w12037] mode=indexing
          shift-right: [w12035] -> w12032
          shift-left: 0 -> [w12036]
          n6232 = Exclusive Or(1:w12036, 2:w12037) -> (0:w12035:i32)
        }
        n6233 = Build Array(w12032) -> (w12031:i32[])
        n6234 = Byte Array To String(unsigned byte array=w12031) -> (string=w12029:string)
        n6235 = Concatenate Strings(w12028, w12029) -> (w12025:string)
        n6236 = VISA Write(VISA resource name=w12024, write buffer=w12025, error in (no error)=w12023) -> (VISA resource name out=w12022:refnum<visa-resource-name>, error out=w12021:errorcluster)  [unwired: 1 out]
      }
      frame 10 {
        n6237 = Multiply(x="Set CT Position:", y=10.0) -> (x*y=w12038:dbl)
        n6238 = To Unsigned Long Integer(number=w12038) -> (unsigned 32bit integer=w12039:u32)
        n6239 = Quotient & Remainder(x=w12039, y=u32 256) -> (x-y*floor(x/y)=w12044:u32, floor(x/y)=w12043:u32)
        n6240 = Build Array(w12044, w12043) -> (w12041:u32[])
        n6241 = Byte Array To String(unsigned byte array=w12041) -> (string=w12051:string)
        n6242 = Concatenate Strings("\nz", w12051) -> (w12052:string)
        n6243 = String To Byte Array(string=w12052) -> (unsigned byte array=w12058:u8[])
        n6244 = for {
          tunnel: w12058 -> [w12061] mode=indexing
          shift-right: [w12059] -> w12056
          shift-left: 0 -> [w12060]
          n6245 = Exclusive Or(1:w12060, 2:w12061) -> (0:w12059:i32)
        }
        n6246 = Build Array(w12056) -> (w12055:i32[])
        n6247 = Byte Array To String(unsigned byte array=w12055) -> (string=w12053:string)
        n6248 = Concatenate Strings(w12052, w12053) -> (w12050:string)
        n6249 = VISA Write(VISA resource name=w12049, write buffer=w12050, error in (no error)=w12048) -> (VISA resource name out=w12047:refnum<visa-resource-name>, error out=w12046:errorcluster)  [unwired: 1 out]
      }
      frame 11 {
        w12069 = "\t\u0003\u0006"
        n6250 = String To Byte Array(string=w12069) -> (unsigned byte array=w12066:u8[])
        n6251 = for {
          tunnel: w12066 -> [w12075] mode=indexing
          shift-right: [w12073] -> w12068
          shift-left: 0 -> [w12074]
          n6252 = Exclusive Or(1:w12074, 2:w12075) -> (0:w12073:i32)
        }
        n6253 = Build Array(w12068) -> (w12070:i32[])
        n6254 = Byte Array To String(unsigned byte array=w12070) -> (string=w12071:string)
        n6255 = Concatenate Strings(w12069, w12071) -> (w12072:string)
        n6256 = VISA Write(VISA resource name=w12065, write buffer=w12072, error in (no error)=w12064) -> (VISA resource name out=w12063:refnum<visa-resource-name>, error out=w12062:errorcluster)  [unwired: 1 out]
      }
      frame 12 {
        w12084 = "\t\u0003\b"
        n6257 = String To Byte Array(string=w12084) -> (unsigned byte array=w12080:u8[])
        n6258 = for {
          tunnel: w12080 -> [w12089] mode=indexing
          shift-right: [w12087] -> w12082
          shift-left: 0 -> [w12088]
          n6259 = Exclusive Or(1:w12088, 2:w12089) -> (0:w12087:i32)
        }
        n6260 = Build Array(w12082) -> (w12083:i32[])
        n6261 = Byte Array To String(unsigned byte array=w12083) -> (string=w12085:string)
        n6262 = Concatenate Strings(w12084, w12085) -> (w12086:string)
        n6263 = VISA Write(VISA resource name=w12079, write buffer=w12086, error in (no error)=w12078) -> (VISA resource name out=w12077:refnum<visa-resource-name>, error out=w12076:errorcluster)  [unwired: 1 out]
      }
      frame 13 {
        w12098 = "\t\u001b\u0000"
        n6264 = String To Byte Array(string=w12098) -> (unsigned byte array=w12094:u8[])
        n6265 = for {
          tunnel: w12094 -> [w12103] mode=indexing
          shift-right: [w12101] -> w12096
          shift-left: 0 -> [w12102]
          n6266 = Exclusive Or(1:w12102, 2:w12103) -> (0:w12101:i32)
        }
        n6267 = Build Array(w12096) -> (w12097:i32[])
        n6268 = Byte Array To String(unsigned byte array=w12097) -> (string=w12099:string)
        n6269 = Concatenate Strings(w12098, w12099) -> (w12100:string)
        n6270 = VISA Write(VISA resource name=w12093, write buffer=w12100, error in (no error)=w12092) -> (VISA resource name out=w12091:refnum<visa-resource-name>, error out=w12090:errorcluster)  [unwired: 1 out]
      }
      frame 14 {
        w12114 = "\t\u001b\u0001"
        n6271 = String To Byte Array(string=w12114) -> (unsigned byte array=w12108:u8[])
        n6272 = for {
          tunnel: w12108 -> [w12117] mode=indexing
          shift-right: [w12115] -> w12110
          shift-left: 0 -> [w12116]
          n6273 = Exclusive Or(1:w12116, 2:w12117) -> (0:w12115:i32)
        }
        n6274 = Build Array(w12110) -> (w12111:i32[])
        n6275 = Byte Array To String(unsigned byte array=w12111) -> (string=w12112:string)
        n6276 = Concatenate Strings(w12114, w12112) -> (w12113:string)
        n6277 = VISA Write(VISA resource name=w12107, write buffer=w12113, error in (no error)=w12106) -> (VISA resource name out=w12105:refnum<visa-resource-name>, error out=w12104:errorcluster)  [unwired: 1 out]
      }
      frame 15 {
        w12126 = "\t\u001b\u0002"
        n6278 = String To Byte Array(string=w12126) -> (unsigned byte array=w12122:u8[])
        n6279 = for {
          tunnel: w12122 -> [w12131] mode=indexing
          shift-right: [w12129] -> w12124
          shift-left: 0 -> [w12130]
          n6280 = Exclusive Or(1:w12130, 2:w12131) -> (0:w12129:i32)
        }
        n6281 = Build Array(w12124) -> (w12125:i32[])
        n6282 = Byte Array To String(unsigned byte array=w12125) -> (string=w12127:string)
        n6283 = Concatenate Strings(w12126, w12127) -> (w12128:string)
        n6284 = VISA Write(VISA resource name=w12121, write buffer=w12128, error in (no error)=w12120) -> (VISA resource name out=w12119:refnum<visa-resource-name>, error out=w12118:errorcluster)  [unwired: 1 out]
      }
      frame 16 {
        w12148 = 256.0 ("y")
        n6285 = Quotient & Remainder(x="Frequency :", y=w12148) -> (x-y*floor(x/y)=w12143:dbl, floor(x/y)=w12147:dbl)
        n6286 = Build Array(w12143) -> (w12144:dbl[])
        n6287 = Quotient & Remainder(x=w12147, y=w12148) -> (x-y*floor(x/y)=w12149:dbl, floor(x/y)=w12153:dbl)
        n6288 = Byte Array To String(unsigned byte array=w12144) -> (string=w12151:string)
        n6289 = Build Array(w12149) -> (w12150:dbl[])
        n6290 = Build Array(w12153) -> (w12145:dbl[])
        n6291 = Byte Array To String(unsigned byte array=w12150) -> (string=w12154:string)
        n6292 = Byte Array To String(unsigned byte array=w12145) -> (string=w12155:string)
        n6293 = Concatenate Strings("\f]", w12151, w12154, w12155, "\u0000" ("string")) -> (w12142:string)
        n6294 = String To Byte Array(string=w12142) -> (unsigned byte array=w12136:u8[])
        n6295 = for {
          tunnel: w12136 -> [w12159] mode=indexing
          shift-right: [w12157] -> w12138
          shift-left: 0 -> [w12158]
          n6296 = Exclusive Or(1:w12158, 2:w12159) -> (0:w12157:i32)
        }
        n6297 = Build Array(w12138) -> (w12139:i32[])
        n6298 = Byte Array To String(unsigned byte array=w12139) -> (string=w12141:string)
        n6299 = Concatenate Strings(w12142, w12141) -> (w12156:string)
        n6300 = VISA Write(VISA resource name=w12135, write buffer=w12156, error in (no error)=w12134) -> (VISA resource name out=w12133:refnum<visa-resource-name>, error out=w12132:errorcluster)  [unwired: 1 out]
      }
      frame 17 {
        n6301 = Build Array("Duty Cycle :") -> (w12173:i8[])
        n6302 = Byte Array To String(unsigned byte array=w12173) -> (string=w12174:string)
        n6303 = Concatenate Strings("\n`", w12174, "\u0000" ("string")) -> (w12170:string)
        n6304 = String To Byte Array(string=w12170) -> (unsigned byte array=w12164:u8[])
        n6305 = for {
          tunnel: w12164 -> [w12178] mode=indexing
          shift-right: [w12176] -> w12166
          shift-left: 0 -> [w12177]
          n6306 = Exclusive Or(1:w12177, 2:w12178) -> (0:w12176:i32)
        }
        n6307 = Build Array(w12166) -> (w12167:i32[])
        n6308 = Byte Array To String(unsigned byte array=w12167) -> (string=w12169:string)
        n6309 = Concatenate Strings(w12170, w12169) -> (w12175:string)
        n6310 = VISA Write(VISA resource name=w12163, write buffer=w12175, error in (no error)=w12162) -> (VISA resource name out=w12161:refnum<visa-resource-name>, error out=w12160:errorcluster)  [unwired: 1 out]
      }
      frame 18 {
        n6311 = flat-sequence {
          frame #0 {
            n6312 = Wait (ms)(milliseconds to wait=u32 100) -> ()  [unwired: 1 out]
          }
          frame #1 {
            n6313 = local write "Ramp Up time_auto"(FALSE ("Ramp Up time_auto")) -> ()
          }
        }
        n6314 = Multiply(x="Ramp up Time:", y=10.0) -> (x*y=w12186:dbl)
        n6315 = To Unsigned Long Integer(number=w12186) -> (unsigned 32bit integer=w12185:u32)
        n6316 = Quotient & Remainder(x=w12185, y=u32 256) -> (x-y*floor(x/y)=w12189:u32, floor(x/y)=w12188:u32)
        n6317 = Build Array(w12189, w12188) -> (w12184:u32[])
        n6318 = Byte Array To String(unsigned byte array=w12184) -> (string=w12192:string)
        n6319 = Concatenate Strings("\n\u001f", w12192) -> (w12193:string)
        n6320 = String To Byte Array(string=w12193) -> (unsigned byte array=w12199:u8[])
        n6321 = for {
          tunnel: w12199 -> [w12204] mode=indexing
          shift-right: [w12202] -> w12197
          shift-left: 0 -> [w12203]
          n6322 = Exclusive Or(1:w12203, 2:w12204) -> (0:w12202:i32)
        }
        n6323 = Build Array(w12197) -> (w12196:i32[])
        n6324 = Byte Array To String(unsigned byte array=w12196) -> (string=w12194:string)
        n6325 = Concatenate Strings(w12193, w12194) -> (w12191:string)
        n6326 = VISA Write(VISA resource name=w12182, write buffer=w12191, error in (no error)=w12181) -> (VISA resource name out=w12180:refnum<visa-resource-name>, error out=w12179:errorcluster)  [unwired: 1 out]
      }
      frame 19 {
        n6327 = Multiply(x="Ramp Down Time :", y=10.0) -> (x*y=w12212:dbl)
        n6328 = flat-sequence {
          frame #0 {
            n6329 = Wait (ms)(milliseconds to wait=u32 100) -> ()  [unwired: 1 out]
          }
          frame #1 {
            n6330 = local write "Ramp Down time_auto"(FALSE ("Ramp Down time_auto")) -> ()
          }
        }
        n6331 = To Unsigned Long Integer(number=w12212) -> (unsigned 32bit integer=w12211:u32)
        n6332 = Quotient & Remainder(x=w12211, y=u32 256) -> (x-y*floor(x/y)=w12215:u32, floor(x/y)=w12214:u32)
        n6333 = Build Array(w12215, w12214) -> (w12210:u32[])
        n6334 = Byte Array To String(unsigned byte array=w12210) -> (string=w12218:string)
        n6335 = Concatenate Strings("\n ", w12218) -> (w12219:string)
        n6336 = String To Byte Array(string=w12219) -> (unsigned byte array=w12225:u8[])
        n6337 = for {
          tunnel: w12225 -> [w12230] mode=indexing
          shift-right: [w12228] -> w12223
          shift-left: 0 -> [w12229]
          n6338 = Exclusive Or(1:w12229, 2:w12230) -> (0:w12228:i32)
        }
        n6339 = Build Array(w12223) -> (w12222:i32[])
        n6340 = Byte Array To String(unsigned byte array=w12222) -> (string=w12220:string)
        n6341 = Concatenate Strings(w12219, w12220) -> (w12217:string)
        n6342 = VISA Write(VISA resource name=w12208, write buffer=w12217, error in (no error)=w12207) -> (VISA resource name out=w12206:refnum<visa-resource-name>, error out=w12205:errorcluster)  [unwired: 1 out]
      }
    }
    n6343 = Not Equal To 0?(x=w11733) -> (x != 0?=w11732:bool)
    n6344 = Concatenate Strings(w11363, w11441) -> (w11434:string)
    n6345 = case shown="True" w11732 {
      tunnel: w11735 -> [w11893 w11903]
      tunnel: w11734 -> [w11892 w11902]
      tunnel: [w11893 w11905] -> w11722
      tunnel: [w11892 w11899] -> w11721
      frame False {
      }
      frame True {
        n6346 = stacked-sequence {
          tunnel: [w11908] -> w11901
          tunnel: w11903 -> [w11908]
          tunnel: [w11907] -> w11900
          tunnel: w11902 -> [w11907]
          frame #0 {
            n6347 = Wait Until Next ms Multiple(millisecond multiple=u32 40) -> ()  [unwired: 1 out]
          }
        }
        n6348 = property class="Instr"(reference=w11901, error in=w11900) -> (reference out=w11898:refnum<visa-resource-name>, error out=w11897:errorcluster, "Serial Settings:Number of Bytes at Serial Port"=w11896:u32)
        n6349 = VISA Read(VISA resource name=w11898, byte count=w11896, error in (no error)=w11897) -> (VISA resource name out=w11895:refnum<visa-resource-name>, error out=w11894:errorcluster)  [unwired: 2 out]
        n6350 = VISA Write(VISA resource name=w11895, write buffer="\u0006", error in (no error)=w11894) -> (VISA resource name out=w11905:refnum<visa-resource-name>, error out=w11899:errorcluster)  [unwired: 1 out]
      }
    }
    n6351 = VISA Write(VISA resource name=w11722, write buffer="\bΞ", error in (no error)=w11721) -> (VISA resource name out=w11727:refnum<visa-resource-name>, error out=w11726:errorcluster)  [unwired: 1 out]
    n6352 = stacked-sequence {
      tunnel: [w11891] -> w11724
      tunnel: w11727 -> [w11891]
      tunnel: [w11890] -> w11723
      tunnel: w11726 -> [w11890]
      frame #0 {
        n6353 = Wait Until Next ms Multiple(millisecond multiple=u32 40) -> ()  [unwired: 1 out]
      }
    }
    n6354 = property class="Instr"(reference=w11724, error in=w11723) -> (reference out=w11728:refnum<visa-resource-name>, error out=w11730:errorcluster, "Serial Settings:Number of Bytes at Serial Port"=w11729:u32)
    n6355 = VISA Read(VISA resource name=w11728, byte count=w11729, error in (no error)=w11730) -> (VISA resource name out=w11372:refnum<visa-resource-name>, read buffer=w11720:string, error out=w11371:errorcluster)  [unwired: 1 out]
    n6356 = Match Pattern(string=w11720, regular expression="¦") -> (after substring=w11368:string)  [unwired: 4 out]
    n6357 = String Length(string=w11368) -> (length=w11719:i32)
    n6358 = String Subset(string=w11368, length (rest)=2 ("length (rest)")) -> (substring=w11717:string)  [unwired: 1 out]
    n6359 = Not Equal To 0?(x=w11719) -> (x != 0?=w11365:bool)
    n6360 = String To Byte Array(string=w11717) -> (unsigned byte array=w11715:u8[])
    n6361 = case shown="True" w11365 {
      tunnel: [w11766 w11770] -> w11370
      tunnel: [w11765 w11769] -> w11369
      tunnel: w11372 -> [w11766 w11768]
      tunnel: w11371 -> [w11765 w11767]
      frame False {
      }
      frame True {
        n6362 = VISA Write(VISA resource name=w11768, write buffer="\u0006", error in (no error)=w11767) -> (VISA resource name out=w11770:refnum<visa-resource-name>, error out=w11769:errorcluster)  [unwired: 1 out]
      }
    }
    n6363 = Index Array(array=w11715, index=1) -> (element=w11711:u8)
    n6364 = Index Array(array=w11715, index=0) -> (element=w11709:u8)
    n6365 = To Unsigned Long Integer(number=w11711) -> (unsigned 32bit integer=w11713:u32)
    n6366 = To Unsigned Long Integer(number=w11709) -> (unsigned 32bit integer=w11708:u32)
    n6367 = Multiply(x=256, y=w11713) -> (x*y=w11710:u32)
    n6368 = Add(x=w11710, y=w11708) -> (x+y=w11459:u32)
    n6369 = case shown="True" w11365 {
      tunnel: w11459 -> [_ w11818]
      frame False {
      }
      frame True {
        "Reflected Power" <- w11818
      }
    }
    n6370 = VISA Write(VISA resource name=w11370, write buffer=w11434, error in (no error)=w11369) -> (VISA resource name out=w11438:refnum<visa-resource-name>, error out=w11437:errorcluster)  [unwired: 1 out]
    n6371 = stacked-sequence {
      tunnel: [w11796] -> w11436
      tunnel: w11438 -> [w11796]
      tunnel: [w11795] -> w11435
      tunnel: w11437 -> [w11795]
      frame #0 {
        n6372 = Wait Until Next ms Multiple(millisecond multiple=u32 40) -> ()  [unwired: 1 out]
      }
    }
    n6373 = property class="Instr"(reference=w11436, error in=w11435) -> (reference out=w11439:refnum<visa-resource-name>, error out=w11440:errorcluster, "Serial Settings:Number of Bytes at Serial Port"=w11364:u32)
    n6374 = VISA Read(VISA resource name=w11439, byte count=w11364, error in (no error)=w11440) -> (VISA resource name out=w11421:refnum<visa-resource-name>, read buffer=w11431:string, error out=w11420:errorcluster)  [unwired: 1 out]